vi "Alyssa_GlueFatLinesV2.vi"(5 "Image Feed":T7=refnum, 7 "Template Path":path=path "C:/Users/Aerotech/Documents/BNL_ThermomechanicalStave/Utils/ConfigurationFiles_and_Templates/1_ModulePlacement", 8 "error in":errorcluster, 9 "um/pix resolution":dbl=1.58, 10 "Module corner coordinates":T3={"X [mm]"=-325.4922095457569, "Y [mm]"=111.42987050829626, "Z [mm] "=34.99996599632762}, 11 "XYZ Stage Control":refnum<k24>) -> (0 "error out":errorcluster={"status"=FALSE, "code"=1073676418, "source"="VISA Close in GlueSingleModule(SubVI).vi->2_VisualizeModulePositioning2.vi->VMP_TestStand.vi"}, 3 "XYZ .NET Refnum out 2":refnum<k24>)   [LabVIEW 2016]
uses:
  C:/Users/Aerotech/Documents/BNLStaveAssembly-blueprint/Bin/Aerotech.A3200.dll
  BNLStaveAssembly-blueprint/Bin/Aerotech.A3200.dll
  <vilib>/vision/Image Controls.llb/IMAQ Image.ctl
  <vilib>/LabVIEW Interface for Arduino/Type Defs/Arduino Resource.ctl
  <vilib>/LabVIEW Interface for Arduino/Type Defs/Board Type.ctl
  <vilib>/LabVIEW Interface for Arduino/Type Defs/Pin Mode.ctl
  <vilib>/LabVIEW Interface for Arduino/LabVIEW Interface for Arduino.lvlib
panel:
  out "mid line speed":cluster{dbl, dbl, dbl}
  out "top/bottom line speed":cluster{dbl, dbl, dbl}
  in  "glue time":dbl=1.83 format="%#_13g"
  out "Module Start":T1
  in  "How many SHORT lines? (actual # will be x2)":i32
  in  "y dist (mm)":dbl
  in  "How many lines? (actual # will be x2)":i32
  out "XYZ .NET Refnum out":refnum<k24>
  in  "?":T2(tab)
  in  "Axis speeds (mm/s)":T4={"vX [mm]"=49.0, "vY [mm]"=49.0, "vZ [mm] "=49.0}
  in  "Home?":bool
  in  "Lowest Z Position":dbl=38.0
  out "Arduino Resource":T5={"VISA resource"="COM4", "Board Type"=enum."Uno", "Connection Type"=enum."USB / Serial", "Bytes Per Packet (15)"=15}
  in  "Digital I/O Pin":u8=7
  in  "Testing?":bool
  out "Difference camera/syringe in X":dbl=-133.03368290747076
  out "Difference camera/syringe in y":dbl=-2.170984960815403
  in  "Path to save collected images":path=path "C:/Users/Aerotech/cernbox/BNL/Stave Assembly Records/2017-06-12/3"
  in  "Estimate distance y":dbl
  in  "Estimate distance x":dbl=130.0
  in  "Lowest Z position Calibration":dbl=17.0
  out "Final Position":T1={"Final X"=-325.49379764644783, "Final Y"=23.533617154160947, "Final Z"=34.99956596392527}
  # "Timers (ms)"
  # "Overview: This takes a pattern of zeroes/ones (.csv file) as well as the start coordinates of the top left corner of a module and places dots of glue  \nRequirements: NI Arduino dependencies\nInstructions: Select a .csv file (ones indicate regions for glue) as well as a starting coordinate (this is default to the top left corner of the module spacer). You \ncan also input axis speeds (default to maximum) and module lengths and widths (default to 90 mm) which are the widths of the module to which you want to \nplace glue. Lastly, one can choose to Home the stage here and can select the lowest position in Z. The default is that the stage moves down 2-3 mm in Z \nwhile dispensing.  The Arduino inputs are default and simply allow the LabView program to drigger the Arduino (which sends a signal to the dispenser). The \nprogram signals to dispense air- all other parameters such as length of dispensing (default: 350 millisec), pressure (default: 48 psi), and vacuum pressure \n(default: 7.8 psi) are set on the dispenser itself. The defaults are highly recommended here."
  # "Positioning Inputs"
  # "Arduino Inputs"
types:
  T1 = cluster{"Final X":dbl, "Final Y":dbl, "Final Z":dbl}
  T2 = enum32{"Instructions and inputs", "Review  and Error Handling"}
  T3 = cluster{"X [mm]":dbl, "Y [mm]":dbl, "Z [mm] ":dbl}
  T4 = cluster{"vX [mm]":dbl, "vY [mm]":dbl, "vZ [mm] ":dbl}
  T5 = typedef "LabVIEW Interface for Arduino.lvlib/Arduino Resource.ctl" = cluster{"VISA resource":refnum<visa-resource-name>, "Board Type":T6, "Connection Type":enum8{"USB / Serial"}, "Bytes Per Packet (15)":u8}
  T6 = typedef "LabVIEW Interface for Arduino.lvlib/Board Type.ctl" = enum16{"Uno", "Dimuelanove w/Atmega 328", "Mega 2560"}
  T7 = typedef "IMAQ Image.ctl" = refnum<image>
  T8 = typedef "LabVIEW Interface for Arduino.lvlib/Pin Mode.ctl" = enum8{"Input", "Output"}
  T9 = cluster{dbl, "Y [mm]":dbl, "Lowest Z Position":dbl}
  T10 = cluster{"Final X":dbl, "Final Y":dbl, "vZ [mm]":dbl}
  T11 = cluster{dbl, "Final Y":dbl, "Lowest Z Position":dbl}
  T12 = cluster{"Final X":dbl, "Final Y":dbl, "Z [mm] ":dbl}
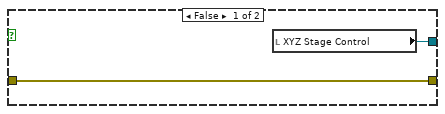
[diagram p2: hidden frame]
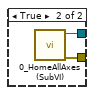
[diagram p3: hidden frame]
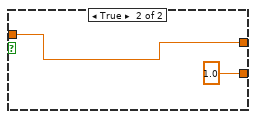
[diagram p5: hidden frame]
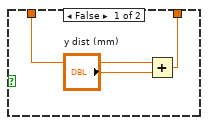
[diagram p6: hidden frame]
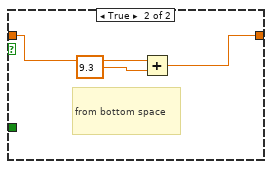
[diagram p7: hidden frame]
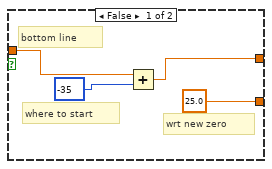
[diagram p11: hidden frame]
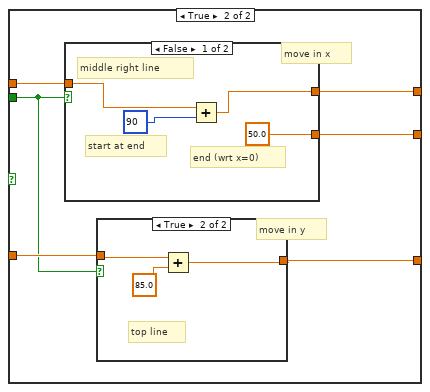
[diagram p12: hidden frame]
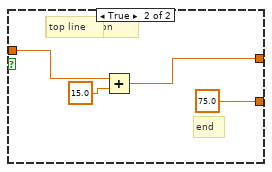
[diagram p13: hidden frame]
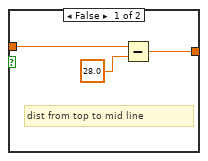
[diagram p14: hidden frame]
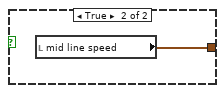
[diagram p15: hidden frame]
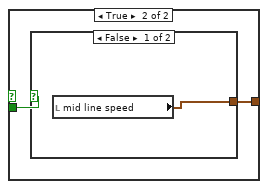
[diagram p16: hidden frame]
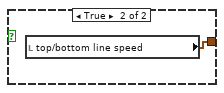
[diagram p17: hidden frame]
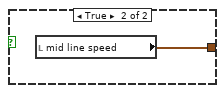
[diagram p18: hidden frame]
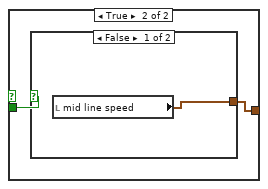
[diagram p19: hidden frame]
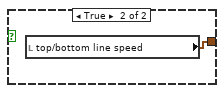
[diagram p20: hidden frame]
diagram:
  n1 = case shown="True" "Testing?" {
    tunnel: [w8 w10] -> w2
    tunnel: [w7 w9] -> w4
    tunnel: "error in" -> [w7 _]
    frame False {
      n2 = local read "XYZ Stage Control"() -> (w8:refnum<k24>)
    }
    frame True {
      n3 = case shown="False" "Home?" {
        tunnel: [w14 w20] -> w10
        tunnel: [w13 w19] -> w9
        frame False {
          w16 = string[] ["X", "Y", "Z"] ("Axes Names")
          n4 = call "Connect.vi"() -> ("error out"=w17:errorcluster, "controller"=w12:refnum<k24>)  [unwired: 10 in]
          n5 = call "EnableMultiple.vi"("error in (no error)"=w17, "axis names"=w16, "controller in"=w12) -> ("error out"=w18:errorcluster, "controller out"=w15:refnum<k24>)  [unwired: 7 in]
          n6 = call "GetCurrentXYZPosition (SubVI).vi"(".NET Refnum in - Device"=w15, "error in (no error)"=w18, "Axes Names"=w16) -> ("error out"=w13:errorcluster, ".NET Refnum out  - Device"=w14:refnum<k24>)  [unwired: 3 in, 4 out]
        }
        frame True {
          n7 = call "0_HomeAllAxes (SubVI).vi"() -> ("error out"=w19:errorcluster, "controller out"=w20:refnum<k24>)  [unwired: 8 in, 2 out]
        }
      }
    }
  }
  n8 = flat-sequence {
    tunnel: [w38] -> w6
    tunnel: w4 -> [w28]
    tunnel: w2 -> [w22]
    tunnel: [w186] -> w1
    tunnel: w6 -> [w192]
    tunnel: w1 -> [w331]
    frame #0 {
      n9 = flat-sequence {
        tunnel: w28 -> [w52]
        tunnel: [w51] -> w23
        tunnel: w22 -> [w45]
        tunnel: w23 -> [w54]
        tunnel: [w53] -> w21
        tunnel: [w73] -> w25
        tunnel: w21 -> [w72]
        tunnel: w25 -> [w134]
        tunnel: [w132] -> w24
        tunnel: [w165] -> w26
        tunnel: w24 -> [w166]
        frame #0 {
          n10 = local read "Module corner coordinates"() -> (w47:T3)
          n11 = Unbundle(w47) -> ("X [mm]"=w44:dbl, "Y [mm]"=w41:dbl)  [unwired: 1 out]
          n12 = local read "Axis speeds (mm/s)"() -> (w50:T4)
          n13 = Add(x=w44, y=133.0) -> (x+y=w42:dbl)
          n14 = Bundle(w42, "Y [mm]"=w41, "Lowest Z Position"="Lowest Z Position") -> (w46:T9)  [unwired: 1 in]
          n15 = Bundle(w42, "Y [mm]"=w41, "Lowest Z Position"="Lowest Z Position") -> (w39:T9)  [unwired: 1 in]
          n16 = call "Go2XYZ (SubVI).vi"(".NET Refnum in"=w45, "Go to Coordinates"=w46, "Axis Speeds"=w50, "error in (no error)"=w52) -> (".NET Refnum out"=w49:refnum<k24>, "Final Position"=→"Final Position":T1, "error out"=w51:errorcluster)  [unwired: 7 in, 2 out]
          n17 = local write "Module corner coordinates"(w39) -> ()
          n18 = local write "XYZ Stage Control"(w49) -> ()
        }
        frame #1 {
          n19 = while {
            tunnel: w54 -> [w71]
            tunnel: [w67] -> w53
            stop <- w70 stop-if-true
            n20 = local read "Module corner coordinates"() -> (w65:T3)
            n21 = call "Lower glue mount"("error in (no error)"=w71) -> ("Move Z down"=w62:dbl, "Move Z up"=w61:dbl, "Accept current Z?"=w70:bool, "error out"=w68:errorcluster)  [unwired: 14 in, 1 out]
            n22 = local read "Lowest Z Position"() -> (w55:dbl)
            n23 = local read "Axis speeds (mm/s)"() -> (w69:T4)
            n24 = local read "XYZ Stage Control"() -> (w57:refnum<k24>)
            n25 = Add(x=w55, y=w62) -> (x+y=w59:dbl)
            n26 = Subtract(x=w59, y=w61) -> (x-y=w58:dbl)
            n27 = Unbundle(w65) -> ("X [mm]"=w64:dbl, "Y [mm]"=w63:dbl)  [unwired: 1 out]
            n28 = Bundle("X [mm]"=w64, "Y [mm]"=w63, w58) -> (w60:cluster{"X [mm]":dbl, "Y [mm]":dbl, dbl})  [unwired: 1 in]
            n29 = local write "Lowest Z Position"(w58) -> ()
            n30 = call "Go2XYZ (SubVI).vi"(".NET Refnum in"=w57, "Go to Coordinates"=w60, "Axis Speeds"=w69, "error in (no error)"=w68) -> (".NET Refnum out"=w66:refnum<k24>, "Final Position"=w56:T1, "error out"=w67:errorcluster)  [unwired: 7 in, 2 out]
            n31 = local write "XYZ Stage Control"(w66) -> ()
            n32 = local write "Final Position"(w56) -> ()
          }
        }
        frame #2 {
          n33 = call "Calibrate distance?"("error in (no error)"=w72) -> ("Calibrate distance?"=w74:bool, "error out"=w75:errorcluster)  [unwired: 16 in, 1 out]
          n34 = case shown="True" w74 {
            tunnel: w75 -> [w76 w78]
            tunnel: [w76 w79] -> w73
            frame False {
            }
            frame True {
              n35 = flat-sequence {
                tunnel: w78 -> [w81]
                tunnel: [w80] -> w77
                frame #0 {
                  n36 = local read "Final Position"() -> (w88:T1)
                  n37 = local read "Axis speeds (mm/s)"() -> (w84:T4)
                  n38 = local read "XYZ Stage Control"() -> (w83:refnum<k24>)
                  n39 = Unbundle(w88) -> ("Final X"=w86:dbl, "Final Y"=w87:dbl)  [unwired: 1 out]
                  n40 = Bundle("Final X"=w86, "Final Y"=w87, "vZ [mm]"=-20.0) -> (w90:T10)  [unwired: 1 in]
                  n41 = call "Go2XYZ (SubVI).vi"(".NET Refnum in"=w83, "Go to Coordinates"=w90, "Axis Speeds"=w84, "error in (no error)"=w81) -> (".NET Refnum out"=w82:refnum<k24>, "Final Position"=w85:T1, "error out"=w80:errorcluster)  [unwired: 7 in, 2 out]
                  n42 = local write "XYZ Stage Control"(w82) -> ()
                  n43 = local write "Final Position"(w85) -> ()
                }
              }
              n44 = while {
                tunnel: [w130] -> w79
                tunnel: w77 -> [w118]
                i -> [w115]
                stop <- w131 stop-if-true
                n45 = local read "Final Position"() -> (w92:T1)
                n46 = Unbundle(w92) -> ("Final X"=w97:dbl, "Final Y"=w95:dbl, "Final Z"=w96:dbl)
                n47 = local read "Testing?"() -> (w113:bool)
                n48 = local read "Axis speeds (mm/s)"() -> (w120:T4)
                n49 = local read "XYZ Stage Control"() -> (w116:refnum<k24>)
                n50 = Subtract(x=w95, y=220.0) -> (x-y=w93:dbl)
                n51 = Equal To 0?(x=w115) -> (x = 0?=w114:bool)
                n52 = And(x=w113, y=w114) -> (x .and. y?=w112:bool)
                n53 = Bundle("Final X"=w97, w93, "Final Z"=w96) -> (w98:cluster{"Final X":dbl, dbl, "Final Z":dbl})  [unwired: 1 in]
                n54 = call "CalibrateDistanceCameraSyringe.vi"("Path to save collected images"="Path to save collected images", "Image Feed"="Image Feed", "Off stave position"=w98, ".NET Refnum in"=w116, "Axis speeds (mm/s)"=w120, "Lowest Z Position"="Lowest Z position Calibration", "Estimate distance y"="Estimate distance y", "um/pix resolution"="um/pix resolution", "Estimate distance x"="Estimate distance x", "Template Path"="Template Path", "error in"=w118, "Testing?"=w112) -> ("XYZ .NET Refnum out"=w119:refnum<k24>, "error out"=w117:errorcluster, "X/Y difference (CAMERA - SYRINGE)"=w127:dbl[][])  [unwired: 1 in]
                n55 = local read "Difference camera/syringe in X"() -> (w102:dbl)
                n56 = local read "Difference camera/syringe in y"() -> (w99:dbl)
                n57 = local read "Lowest Z position Calibration"() -> (w104:dbl)
                n58 = call "Accept calibration?"("error in (no error)"=w117) -> ("Change in lowest Z"=w106:dbl, "Change in distance Y estimate"=w107:dbl, "Change in distance X estimate"=w108:dbl, "Accept the distance syringe/camera?"=w131:bool, "error out"=w130:errorcluster)  [unwired: 13 in, 1 out]
                n59 = local write "XYZ Stage Control"(w119) -> ()
                n60 = Index Array(array=w127, index (row) #1=0 ("index (row)"), index (col) #1=0 ("disabled index (col)"), index (row) #2=0 ("index (row)"), index (col) #2=1 ("disabled index (col)")) -> (element #1=→"Difference camera/syringe in X":dbl, element #2=→"Difference camera/syringe in y":dbl)
                n61 = Add(x=w102, y=w108) -> (x+y=w101:dbl)
                n62 = Add(x=w99, y=w107) -> (x+y=w100:dbl)
                n63 = Add(x=w104, y=w106) -> (x+y=w105:dbl)
                n64 = local write "Difference camera/syringe in X"(w101) -> ()
                n65 = local write "Difference camera/syringe in y"(w100) -> ()
                n66 = local write "Lowest Z position Calibration"(w105) -> ()
              }
            }
          }
        }
        frame #3 {
          n67 = flat-sequence {
            tunnel: w134 -> [w141]
            tunnel: [w138] -> w133
            tunnel: [w152] -> w132
            tunnel: w133 -> [w153]
            frame #0 {
              n68 = local read "Module corner coordinates"() -> (w151:T3)
              n69 = local read "Difference camera/syringe in y"() -> (w146:dbl)
              n70 = local read "Difference camera/syringe in X"() -> (w147:dbl)
              n71 = Unbundle By Name(w151) -> ("X [mm]"=w137:dbl, "Y [mm]"=w150:dbl)  [unwired: 1 out]
              n72 = Subtract(x=w150, y=w146) -> (x-y=w148:dbl)
              n73 = Subtract(x=w137, y=133.0) -> (x-y=w135:dbl)
              n74 = local read "Axis speeds (mm/s)"() -> (w142:T4)
              n75 = local read "XYZ Stage Control"() -> (w143:refnum<k24>)
              n76 = Subtract(x=w135, y=w147) -> (x-y=w149:dbl)
              n77 = Bundle(w149, w148, "index (row)"=-20.0) -> (w140:cluster{dbl, dbl, "index (row)":dbl})  [unwired: 1 in]
              n78 = call "Go2XYZ (SubVI).vi"(".NET Refnum in"=w143, "Go to Coordinates"=w140, "Axis Speeds"=w142, "error in (no error)"=w141) -> (".NET Refnum out"=w144:refnum<k24>, "Final Position"=w145:T1, "error out"=w138:errorcluster)  [unwired: 7 in, 2 out]
              n79 = local write "XYZ Stage Control"(w144) -> ()
              n80 = local write "Module corner coordinates"(w145) -> ()
            }
            frame #1 {
              n81 = local read "Module corner coordinates"() -> (w158:T3)
              n82 = local read "Lowest Z Position"() -> (w161:dbl)
              n83 = local read "Axis speeds (mm/s)"() -> (w155:T4)
              n84 = local read "XYZ Stage Control"() -> (w154:refnum<k24>)
              n85 = Unbundle(w158) -> ("X [mm]"=w159:dbl, "Y [mm]"=w160:dbl)  [unwired: 1 out]
              n86 = Subtract(x=w161, y=2.0) -> (x-y=w163:dbl)
              n87 = Bundle("X [mm]"=w159, "Y [mm]"=w160, w163) -> (w164:cluster{"X [mm]":dbl, "Y [mm]":dbl, dbl})  [unwired: 1 in]
              n88 = call "Go2XYZ (SubVI).vi"(".NET Refnum in"=w154, "Go to Coordinates"=w164, "Axis Speeds"=w155, "error in (no error)"=w153) -> (".NET Refnum out"=w156:refnum<k24>, "Final Position"=w157:T1, "error out"=w152:errorcluster)  [unwired: 7 in, 2 out]
              n89 = local write "XYZ Stage Control"(w156) -> ()
              n90 = local write "Module corner coordinates"(w157) -> ()
            }
          }
        }
        frame #4 {
          n91 = while {
            tunnel: w166 -> [w180]
            tunnel: [w182] -> w165
            stop <- w167 continue-if-true
            n92 = local read "Module corner coordinates"() -> (w179:T3)
            n93 = call "Ready to glue?"("error in (no error)"=w180) -> ("Move in Z"=w176:dbl, "Move in Y"=w177:dbl, "Move in X"=w178:dbl, "Oh yeah! Reset Arduino and go!"=w167:bool, "error out"=w181:errorcluster)  [unwired: 13 in, 1 out]
            n94 = local read "Axis speeds (mm/s)"() -> (w185:T4)
            n95 = local read "XYZ Stage Control"() -> (w183:refnum<k24>)
            n96 = Unbundle(w179) -> ("X [mm]"=w175:dbl, "Y [mm]"=w174:dbl, "Z [mm]"=w173:dbl)
            n97 = Add(x=w175, y=w178) -> (x+y=w170:dbl)
            n98 = Add(x=w174, y=w177) -> (x+y=w172:dbl)
            n99 = Add(x=w173, y=w176) -> (x+y=w171:dbl)
            n100 = Bundle(w170, w172, w171) -> (w169:cluster{dbl, dbl, dbl})  [unwired: 1 in]
            n101 = call "Go2XYZ (SubVI).vi"(".NET Refnum in"=w183, "Go to Coordinates"=w169, "Axis Speeds"=w185, "error in (no error)"=w181) -> (".NET Refnum out"=w184:refnum<k24>, "Final Position"=w168:T1, "error out"=w182:errorcluster)  [unwired: 7 in, 2 out]
            "Module Start" <- w168
            n102 = local write "XYZ Stage Control"(w184) -> ()
            n103 = local write "Final Position"(w168) -> ()
            n104 = local write "Module corner coordinates"(w168) -> ()
          }
        }
      }
      n105 = local read "Digital I/O Pin"() -> (w27:u8)
      n106 = call <vilib>:"Init.vi"("VISA resource"=refnum<visa-resource-name> "GlueCTRL", "error in"=w26) -> ("Arduino Resource"=w30:T5, "error out"=w31:errorcluster)  [unwired: 16 in]
      "Arduino Resource" <- w30
      n107 = call <vilib>:"Set Digital Pin Mode.vi"("Arduino Resource"=w30, "Digital I/O Pin"="Digital I/O Pin", "Pin Mode (Input)"=Pin_Mode."Output", "error in"=w31) -> ("Arduino Resource"=w34:T5, "error out"=w35:errorcluster)  [unwired: 10 in]
      n108 = call <vilib>:"Digital Write Pin.vi"("Arduino Resource"=w34, "Digital I/O Pin (0)"=w27, "Value (0)"=u8 0, "error in"=w35) -> ("Arduino Resource"=w29:T5, "error out"=w38:errorcluster)  [unwired: 10 in]
      n109 = local write "Arduino Resource"(w29) -> ()
    }
    frame #1 {
      n110 = local read "Module Start"() -> (w191:T1)
      n111 = Unbundle By Name(w191) -> ("Final X"=w189:dbl, "Final Y"=w188:dbl, "Final Z"=w187:dbl)
      n112 = for {
        N: "How many lines? (actual # will be x2)" -> [_]
        tunnel: w192 -> [w206]
        tunnel: [w205] -> w186
        shift-right: [w203] -> _
        shift-left: w188 -> [w204]
        tunnel: w187 -> [w202]
        shift-right: [w201] -> _
        shift-left: w189 -> [w200]
        i -> [w195]
        n113 = local read "How many lines? (actual # will be x2)"() -> (w198:i32)
        n114 = Subtract(x=w198, y=2) -> (x-y=w196:i32)
        n115 = Equal?(x=w195, y=w196) -> (x = y?=w193:bool)
        n116 = Equal To 0?(x=w195) -> (x = 0?=w194:bool)
        n117 = for {
          N: 2 -> [_]
          tunnel: w206 -> [w228]
          tunnel: [w226] -> w205
          shift-right: [w225] -> w203
          shift-left: w204 -> [w215]
          tunnel: w194 -> [w216]
          tunnel: w202 -> [w214]
          tunnel: w200 -> [w217]
          tunnel: [w212] -> w201
          tunnel: w193 -> [w207]
          i -> [w213]
          n118 = flat-sequence {
            tunnel: w228 -> [w246]
            tunnel: [w237] -> w223
            tunnel: [w246] -> w222
            tunnel: [w238] -> w221
            tunnel: [w236] -> w220
            tunnel: [w240] -> w219
            tunnel: [w238] -> w218
            tunnel: w217 -> [w235]
            tunnel: w216 -> [w234]
            tunnel: w215 -> [w241]
            tunnel: w214 -> [w240]
            tunnel: w213 -> [w239]
            tunnel: w207 -> [w233]
            tunnel: [w274] -> w210
            tunnel: [w275] -> w209
            tunnel: [w276] -> w208
            tunnel: w218 -> [w276]
            tunnel: w219 -> [w271]
            tunnel: w220 -> [w273]
            tunnel: w221 -> [w272]
            tunnel: w222 -> [w267]
            tunnel: w223 -> [w274]
            tunnel: [w290] -> w230
            tunnel: [w289] -> w229
            tunnel: [w288] -> w227
            tunnel: [w280] -> w224
            tunnel: w210 -> [w278]
            tunnel: w209 -> [w277]
            tunnel: w208 -> [w280]
            tunnel: [w278] -> w211
            tunnel: [w310] -> w226
            tunnel: w227 -> [w295]
            tunnel: w229 -> [w309]
            tunnel: w230 -> [w307]
            tunnel: [w294] -> w225
            tunnel: w224 -> [w294]
            tunnel: [w293] -> w212
            tunnel: w211 -> [w293]
            frame #0 {
              # "line length"
              n119 = Equal To 0?(x=w239) -> (x = 0?=w232:bool)
              n120 = And(x=w232, y=w234) -> (x .and. y?=w245:bool)
              n121 = And(x=w232, y=w233) -> (x .and. y?=w231:bool)
              n122 = case shown="False" w232 {
                tunnel: [0.0 1.0] -> w244
                tunnel: [w248 w251] -> w236
                tunnel: w235 -> [w249 w251]
                frame False {
                  # "start @ end of line"
                  n123 = Add(x=w249, y=90 ("x")) -> (x+y=w248:dbl)
                }
                frame True {
                }
              }
              n124 = case shown="False" w245 {
                tunnel: w241 -> [w254 w264]
                tunnel: [w255 w263] -> w238
                tunnel: w231 -> [w253 _]
                frame False {
                  n125 = case shown="True" w253 {
                    tunnel: [w258 w259] -> w255
                    tunnel: w254 -> [w256 w261]
                    frame False {
                      n126 = Add(x=w256, y="y dist (mm)") -> (x+y=w258:dbl)
                    }
                    frame True {
                      # "center space"
                      n127 = Add(x=w261, y=13.0) -> (x+y=w259:dbl)
                    }
                  }
                }
                frame True {
                  # "from bottom space"
                  n128 = Add(x=w264, y=9.3) -> (x+y=w263:dbl)
                }
              }
              n129 = Multiply(x=90, y=w244) -> (x*y=w243:dbl)
              n130 = Add(x=w235, y=w243) -> (x+y=w237:dbl)
            }
            frame #1 {
              n131 = local read "Axis speeds (mm/s)"() -> (w269:T4)
              n132 = local read "XYZ Stage Control"() -> (w266:refnum<k24>)
              n133 = Bundle("Final X"=w273, w272, "Final Z"=w271) -> (w270:cluster{"Final X":dbl, dbl, "Final Z":dbl})  [unwired: 1 in]
              n134 = call "Go2XYZ (SubVI).vi"(".NET Refnum in"=w266, "Go to Coordinates"=w270, "Axis Speeds"=w269, "error in (no error)"=w267) -> (".NET Refnum out"=w265:refnum<k24>, "Final Position"=w268:T1, "error out"=w275:errorcluster)  [unwired: 7 in, 2 out]
              n135 = local write "XYZ Stage Control"(w265) -> ()
              n136 = local write "Final Position"(w268) -> ()
            }
            frame #2 {
              n137 = local read "Final Position"() -> (w281:T1)
              n138 = local read "Arduino Resource"() -> (w291:T5)
              n139 = local read "Lowest Z Position"() -> (w287:dbl)
              n140 = local read "Digital I/O Pin"() -> (w290:u8)
              n141 = local read "Axis speeds (mm/s)"() -> (w284:T4)
              n142 = local read "XYZ Stage Control"() -> (w285:refnum<k24>)
              n143 = Unbundle(w281) -> ("Final Y"=w279:dbl)  [unwired: 2 out]
              n144 = Bundle(w278, "Final Y"=w279, "Lowest Z Position"=w287) -> (w283:T11)  [unwired: 1 in]
              n145 = call <vilib>:"Digital Write Pin.vi"("Arduino Resource"=w291, "Digital I/O Pin (0)"=w290, "Value (0)"=u8 1, "error in"=w277) -> ("Arduino Resource"=w289:T5, "error out"=w288:errorcluster)  [unwired: 10 in]
              n146 = call "Go2XYZ (SubVI).vi"(".NET Refnum in"=w285, "Go to Coordinates"=w283, "Axis Speeds"=w284) -> (".NET Refnum out"=w286:refnum<k24>, "Final Position"=w282:T1)  [unwired: 8 in, 3 out]
              n147 = local write "Arduino Resource"(w289) -> ()
              n148 = local write "XYZ Stage Control"(w286) -> ()
              n149 = local write "Final Position"(w282) -> ()
            }
            frame #3 {
              n150 = local read "Module corner coordinates"() -> (w304:T3)
              n151 = call <vilib>:"Digital Write Pin.vi"("Arduino Resource"=w309, "Digital I/O Pin (0)"=w307, "Value (0)"=u8 0, "error in"=w295) -> ("Arduino Resource"=w306:T5, "error out"=w310:errorcluster)  [unwired: 10 in]
              n152 = local write "Arduino Resource"(w306) -> ()
              n153 = local read "Final Position"() -> (w305:T1)
              n154 = local read "Axis speeds (mm/s)"() -> (w299:T4)
              n155 = local read "XYZ Stage Control"() -> (w298:refnum<k24>)
              n156 = Unbundle(w305) -> ("Final X"=w303:dbl, "Final Y"=w302:dbl)  [unwired: 1 out]
              n157 = Unbundle(w304) -> ("Z [mm]"=w301:dbl)  [unwired: 2 out]
              n158 = Bundle("Final X"=w303, "Final Y"=w302, "Z [mm]"=w301) -> (w300:T12)  [unwired: 1 in]
              n159 = call "Go2XYZ (SubVI).vi"(".NET Refnum in"=w298, "Go to Coordinates"=w300, "Axis Speeds"=w299) -> (".NET Refnum out"=→"XYZ .NET Refnum out":refnum<k24>, "Final Position"=w297:T1)  [unwired: 8 in, 3 out]
              n160 = local write "Final Position"(w297) -> ()
            }
          }
        }
      }
    }
    frame #2 {
      n161 = local read "Module Start"() -> (w332:T1)
      n162 = Unbundle By Name(w332) -> ("Final X"=w319:dbl, "Final Y"=w320:dbl, "Final Z"=w329:dbl)
      n163 = local read "glue time"() -> (w315:dbl)
      n164 = Divide(x=40.0 ("vX [mm]"), y=w315) -> (x/y=w313:dbl)
      n165 = Divide(x=60.0 ("vX [mm]"), y="glue time") -> (x/y=w314:dbl)
      n166 = for {
        N: "How many SHORT lines? (actual # will be x2)" -> [_]
        tunnel: w331 -> [w350]
        tunnel: [w349] -> w323
        shift-right: [w347] -> _
        shift-left: w320 -> [w348]
        tunnel: w329 -> [w346]
        shift-right: [w345] -> _
        shift-left: w319 -> [w344]
        i -> [w339]
        n167 = local read "How many SHORT lines? (actual # will be x2)"() -> (w342:i32)
        n168 = Subtract(x=w342, y=1) -> (x-y=w340:i32)
        n169 = Equal?(x=w339, y=w340) -> ()  [unwired: 1 out]
        n170 = Equal To 0?(x=w339) -> (x = 0?=w338:bool)
        n171 = for {
          N: 2 -> [_]
          tunnel: w350 -> [w377]
          tunnel: [w375] -> w349
          shift-right: [w374] -> w347
          shift-left: w348 -> [w366]
          tunnel: w338 -> [w357]
          tunnel: w346 -> [w365]
          tunnel: w344 -> [w358]
          tunnel: [w363] -> w345
          i -> [w364]
          n172 = flat-sequence {
            tunnel: w377 -> [w390]
            tunnel: [w385] -> w372
            tunnel: [w390] -> w371
            tunnel: [w386] -> w370
            tunnel: [w384] -> w369
            tunnel: [w388] -> w368
            tunnel: [w386] -> w367
            tunnel: w358 -> [w383]
            tunnel: w357 -> [w381]
            tunnel: w366 -> [w389]
            tunnel: w365 -> [w388]
            tunnel: w364 -> [w387]
            tunnel: [w380] -> w356
            tunnel: [w380] -> w354
            tunnel: [w443] -> w361
            tunnel: [w442] -> w360
            tunnel: [w441] -> w359
            tunnel: w367 -> [w441]
            tunnel: w368 -> [w438]
            tunnel: w369 -> [w440]
            tunnel: w370 -> [w439]
            tunnel: w371 -> [w435]
            tunnel: w372 -> [w443]
            tunnel: w357 -> [w429]
            tunnel: w356 -> [w431]
            tunnel: [w430] -> w355
            tunnel: w354 -> [w430]
            tunnel: [w429] -> w352
            tunnel: [w467] -> w379
            tunnel: [w466] -> w378
            tunnel: [w465] -> w376
            tunnel: [w458] -> w373
            tunnel: w361 -> [w456]
            tunnel: w360 -> [w455]
            tunnel: w359 -> [w458]
            tunnel: [w456] -> w362
            tunnel: w355 -> [w453]
            tunnel: [w453] -> w353
            tunnel: w352 -> [w452]
            tunnel: [w452] -> w351
            tunnel: [w497] -> w375
            tunnel: w376 -> [w484]
            tunnel: w378 -> [w480]
            tunnel: w379 -> [w495]
            tunnel: [w483] -> w374
            tunnel: w373 -> [w483]
            tunnel: [w482] -> w363
            tunnel: w362 -> [w482]
            tunnel: w353 -> [w479]
            tunnel: w351 -> [w478]
            frame #0 {
              # "where to move"
              n173 = Equal To 0?(x=w387) -> (x = 0?=w380:bool)
              n174 = case shown="False" w381 {
                tunnel: w389 -> [w392 w414]
                tunnel: [w391 w413] -> w386
                tunnel: [w395 w412] -> w384
                tunnel: w383 -> [w396 w411]
                tunnel: [w394 w410] -> w382
                tunnel: w380 -> [w393 w409]
                frame False {
                  # "move in y"
                  # "move in x"
                  n175 = case shown="True" w393 {
                    tunnel: [w403 w407] -> w395
                    tunnel: w396 -> [w404 w408]
                    tunnel: [25.0 -50.0 ("y")] -> w394
                    frame False {
                      # "bottom line"
                      # "wrt new zero"
                      # "where to start"
                      n176 = Add(x=w404, y=-35 ("x")) -> (x+y=w403:dbl)
                    }
                    frame True {
                      # "middle left"
                      # "end wrt previous x"
                      # "where to start"
                      n177 = Subtract(x=w408, y=10.0) -> (x-y=w407:dbl)
                    }
                  }
                  n178 = case shown="False" w393 {
                    tunnel: w392 -> [w398 w400]
                    tunnel: [w399 w400] -> w391
                    frame False {
                      # "dist to bottom from middle"
                      n179 = Subtract(x=w398, y=53.0) -> (x-y=w399:dbl)
                    }
                    frame True {
                      # "stay mid line"
                    }
                  }
                }
                frame True {
                  # "move in y"
                  # "move in x"
                  n180 = case shown="False" w409 {
                    tunnel: [w417 w421] -> w412
                    tunnel: w411 -> [w418 w422]
                    tunnel: [50.0 75.0 ("y")] -> w410
                    frame False {
                      # "middle right line"
                      # "end (wrt x=0)"
                      # "start at end"
                      n181 = Add(x=w418, y=90 ("x")) -> (x+y=w417:dbl)
                    }
                    frame True {
                      # "end"
                      # "top line"
                      # "start position"
                      n182 = Add(x=w422, y=15.0) -> (x+y=w421:dbl)
                    }
                  }
                  n183 = case shown="True" w409 {
                    tunnel: w414 -> [w424 w426]
                    tunnel: [w425 w427] -> w413
                    frame False {
                      # "dist from top to mid line"
                      n184 = Subtract(x=w424, y=28.0) -> (x-y=w425:dbl)
                    }
                    frame True {
                      # "top line"
                      n185 = Add(x=w426, y=85.0) -> (x+y=w427:dbl)
                    }
                  }
                }
              }
              n186 = Add(x=w383, y=w382) -> (x+y=w385:dbl)
            }
            frame #1 {
              n187 = case shown="False" w429 {
                tunnel: [w445 w449] -> w432
                tunnel: w431 -> [w444 w448]
                frame False {
                  n188 = case shown="False" w444 {
                    tunnel: [w446 w447] -> w445
                    frame False {
                      n189 = local read "top/bottom line speed"() -> (w446:cluster{dbl, dbl, dbl})
                    }
                    frame True {
                      n190 = local read "mid line speed"() -> (w447:cluster{dbl, dbl, dbl})
                    }
                  }
                }
                frame True {
                  n191 = case shown="False" w448 {
                    tunnel: [w450 w451] -> w449
                    frame False {
                      n192 = local read "mid line speed"() -> (w450:cluster{dbl, dbl, dbl})
                    }
                    frame True {
                      n193 = local read "top/bottom line speed"() -> (w451:cluster{dbl, dbl, dbl})
                    }
                  }
                }
              }
              n194 = local read "XYZ Stage Control"() -> (w434:refnum<k24>)
              n195 = Bundle(w440, "Final Y"=w439, "Final Z"=w438) -> (w437:cluster{dbl, "Final Y":dbl, "Final Z":dbl})  [unwired: 1 in]
              n196 = call "Go2XYZ (SubVI).vi"(".NET Refnum in"=w434, "Go to Coordinates"=w437, "Axis Speeds"=w432, "error in (no error)"=w435) -> (".NET Refnum out"=w433:refnum<k24>, "Final Position"=w436:T1, "error out"=w442:errorcluster)  [unwired: 7 in, 2 out]
              n197 = local write "XYZ Stage Control"(w433) -> ()
              n198 = local write "Final Position"(w436) -> ()
            }
            frame #2 {
              n199 = local read "Final Position"() -> (w459:T1)
              n200 = case shown="False" w452 {
                tunnel: [w471 w475] -> w454
                tunnel: w453 -> [w470 w474]
                frame False {
                  n201 = case shown="False" w470 {
                    tunnel: [w472 w473] -> w471
                    frame False {
                      n202 = local read "top/bottom line speed"() -> (w472:cluster{dbl, dbl, dbl})
                    }
                    frame True {
                      n203 = local read "mid line speed"() -> (w473:cluster{dbl, dbl, dbl})
                    }
                  }
                }
                frame True {
                  n204 = case shown="False" w474 {
                    tunnel: [w476 w477] -> w475
                    frame False {
                      n205 = local read "mid line speed"() -> (w476:cluster{dbl, dbl, dbl})
                    }
                    frame True {
                      n206 = local read "top/bottom line speed"() -> (w477:cluster{dbl, dbl, dbl})
                    }
                  }
                }
              }
              n207 = local read "Arduino Resource"() -> (w468:T5)
              n208 = local read "Lowest Z Position"() -> (w464:dbl)
              n209 = local read "Digital I/O Pin"() -> (w467:u8)
              n210 = local read "XYZ Stage Control"() -> (w462:refnum<k24>)
              n211 = Unbundle(w459) -> ("Final Y"=w457:dbl)  [unwired: 2 out]
              n212 = Bundle(w456, "Final Y"=w457, "Lowest Z Position"=w464) -> (w461:T11)  [unwired: 1 in]
              n213 = call <vilib>:"Digital Write Pin.vi"("Arduino Resource"=w468, "Digital I/O Pin (0)"=w467, "Value (0)"=u8 1, "error in"=w455) -> ("Arduino Resource"=w466:T5, "error out"=w465:errorcluster)  [unwired: 10 in]
              n214 = call "Go2XYZ (SubVI).vi"(".NET Refnum in"=w462, "Go to Coordinates"=w461, "Axis Speeds"=w454) -> (".NET Refnum out"=w463:refnum<k24>, "Final Position"=w460:T1)  [unwired: 8 in, 3 out]
              n215 = local write "Arduino Resource"(w466) -> ()
              n216 = local write "XYZ Stage Control"(w463) -> ()
              n217 = local write "Final Position"(w460) -> ()
            }
            frame #3 {
              n218 = local read "Module Start"() -> (w492:T1)
              n219 = call <vilib>:"Digital Write Pin.vi"("Arduino Resource"=w480, "Digital I/O Pin (0)"=w495, "Value (0)"=u8 0, "error in"=w484) -> ("Arduino Resource"=w494:T5, "error out"=w497:errorcluster)  [unwired: 10 in]
              n220 = local read "Final Position"() -> (w493:T1)
              n221 = local write "Arduino Resource"(w494) -> ()
              n222 = local read "XYZ Stage Control"() -> (w487:refnum<k24>)
              n223 = case shown="True" w478 {
                tunnel: [w499 w503] -> w481
                tunnel: w479 -> [w498 w502]
                frame False {
                  n224 = case shown="False" w498 {
                    tunnel: [w500 w501] -> w499
                    frame False {
                      n225 = local read "top/bottom line speed"() -> (w500:cluster{dbl, dbl, dbl})
                    }
                    frame True {
                      n226 = local read "mid line speed"() -> (w501:cluster{dbl, dbl, dbl})
                    }
                  }
                }
                frame True {
                  n227 = case shown="True" w502 {
                    tunnel: [w504 w505] -> w503
                    frame False {
                      n228 = local read "mid line speed"() -> (w504:cluster{dbl, dbl, dbl})
                    }
                    frame True {
                      n229 = local read "top/bottom line speed"() -> (w505:cluster{dbl, dbl, dbl})
                    }
                  }
                }
              }
              n230 = Unbundle(w493) -> ("Final X"=w491:dbl, "Final Y"=w490:dbl)  [unwired: 1 out]
              n231 = Unbundle(w492) -> ("Final Z"=w489:dbl)  [unwired: 2 out]
              n232 = Bundle("Final X"=w491, "Final Y"=w490, "Final Z"=w489) -> (w488:T1)  [unwired: 1 in]
              n233 = call "Go2XYZ (SubVI).vi"(".NET Refnum in"=w487, "Go to Coordinates"=w488, "Axis Speeds"=w481) -> (".NET Refnum out"=→"XYZ .NET Refnum out 2":refnum<k24>, "Final Position"=w486:T1)  [unwired: 8 in, 3 out]
              n234 = local write "Final Position"(w486) -> ()
            }
          }
        }
      }
      n235 = Bundle(w313, w313, w313) -> (→"mid line speed":cluster{dbl, dbl, dbl})  [unwired: 1 in]
      n236 = Bundle(w314, w314, w314) -> (→"top/bottom line speed":cluster{dbl, dbl, dbl})  [unwired: 1 in]
      n237 = disable-structure shown="Disabled" {
        frame Disabled {
          n238 = case shown="True" {
            selector: _ -> [_ _]
            tunnel: [_ w333] -> _
            tunnel: _ -> [_ w336]
            frame False {
            }
            frame True {
              # "get back to top"
              n239 = local read "y dist (mm)"() -> (w337:dbl)
              n240 = Add(x=w336, y=w337) -> (x+y=w335:dbl)
              n241 = Add(x=w335, y=73.0) -> (x+y=w333:dbl)
            }
          }
        }
        frame Enabled {
        }
      }
      n242 = local read "Arduino Resource"() -> (w322:T5)
      n243 = local read "Digital I/O Pin"() -> (w321:u8)
      n244 = call <vilib>:"Digital Write Pin.vi"("Arduino Resource"=w322, "Digital I/O Pin (0)"=w321, "error in"=w323) -> ("Arduino Resource"=w327:T5, "error out"=w326:errorcluster)  [unwired: 11 in]
      n245 = call <vilib>:"Close.vi"("Arduino Resource"=w327, "error in"=w326) -> ("error out"=w325:errorcluster)  [unwired: 13 in]
      n246 = VISA Close(VISA resource name=refnum<visa-resource-name> "COM3", error in (no error)=w325) -> (error out=→"error out":errorcluster)
    }
  }
